vi "SMain.vi"() -> ()   [LabVIEW 2011] (continued)
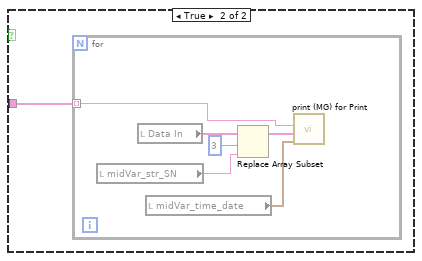
[diagram p4: hidden frame]
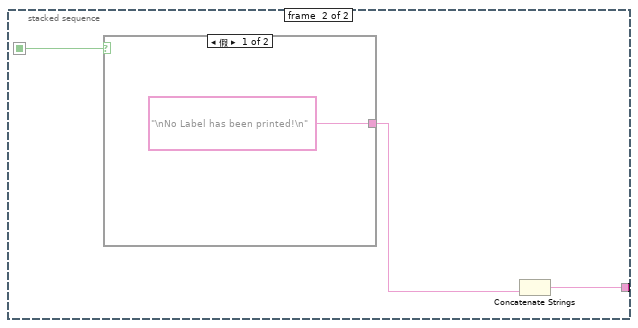
[diagram p5: hidden frame]
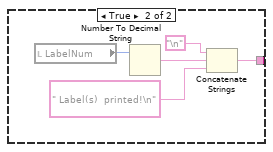
[diagram p6: hidden frame]
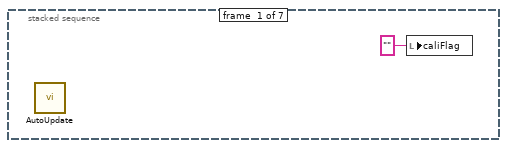
[diagram p8: hidden frame]
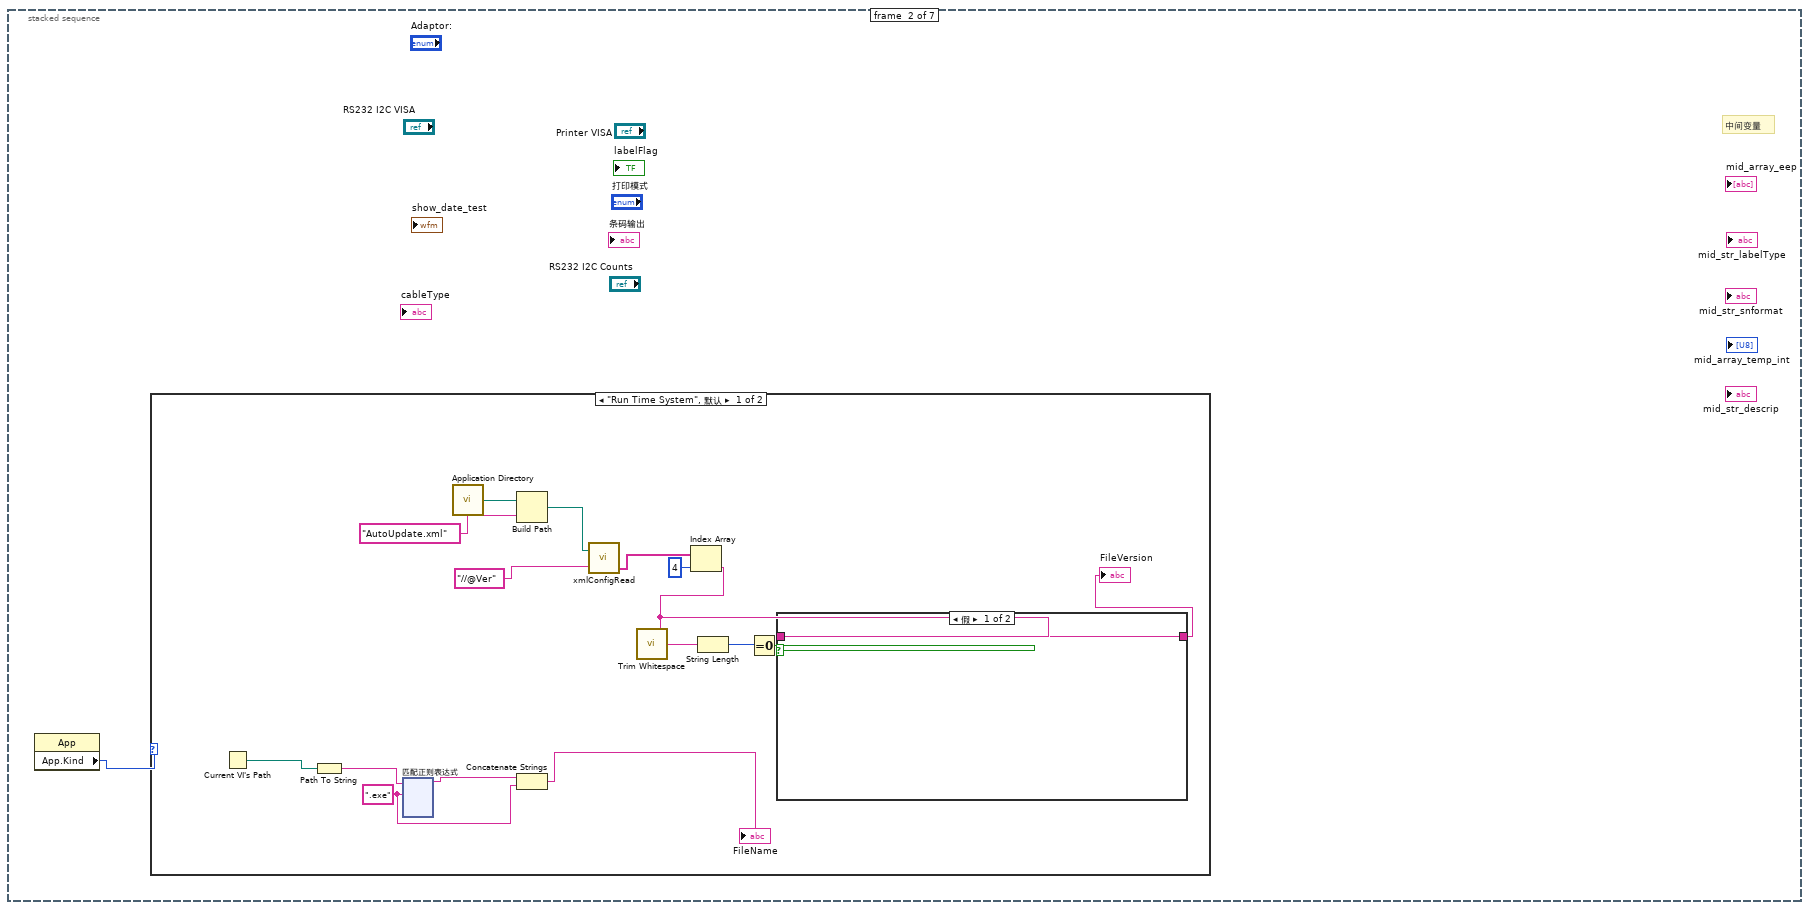
[diagram p9: hidden frame]
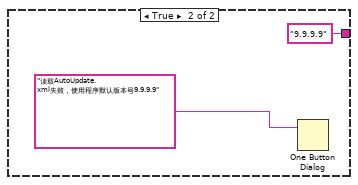
[diagram p10: hidden frame]
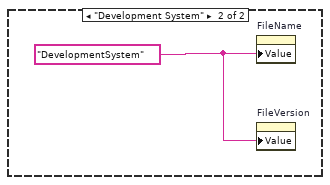
[diagram p11: hidden frame]
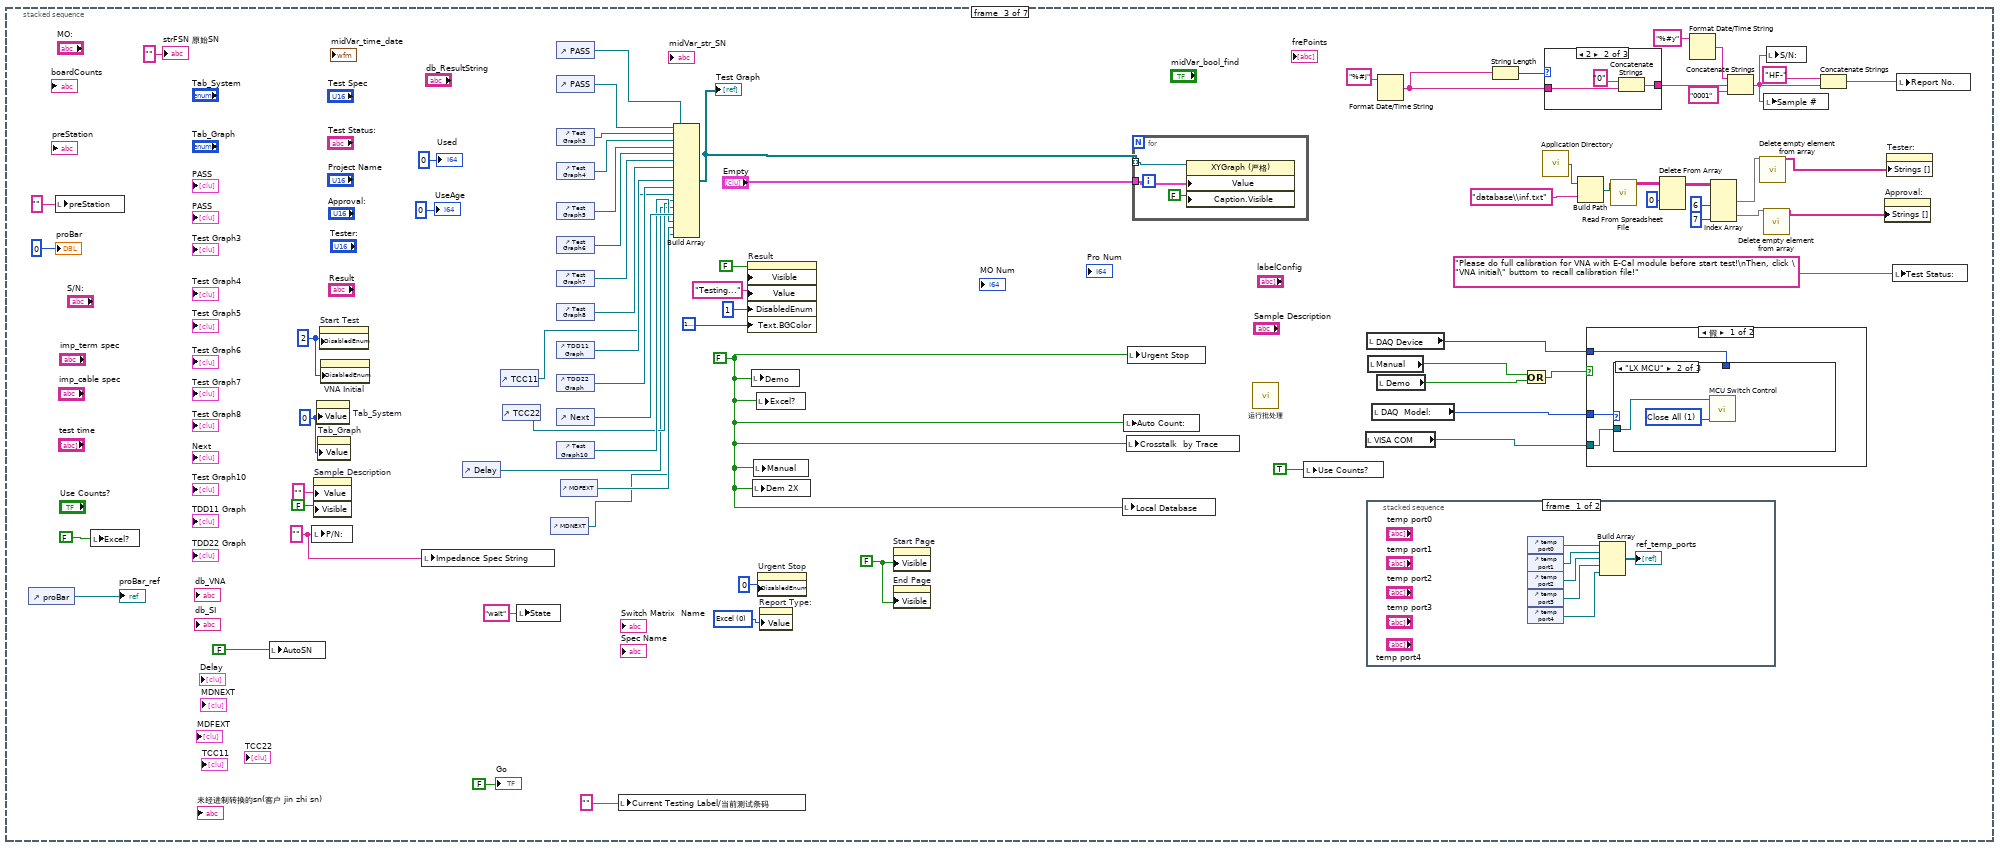
[diagram p12: hidden frame]
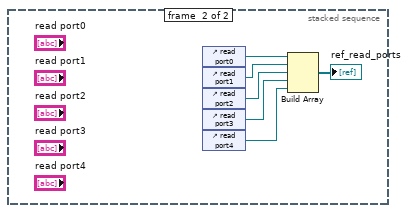
[diagram p13: hidden frame]
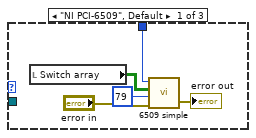
[diagram p14: hidden frame]
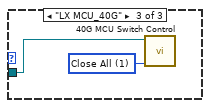
[diagram p15: hidden frame]
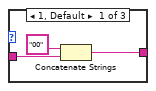
[diagram p17: hidden frame]
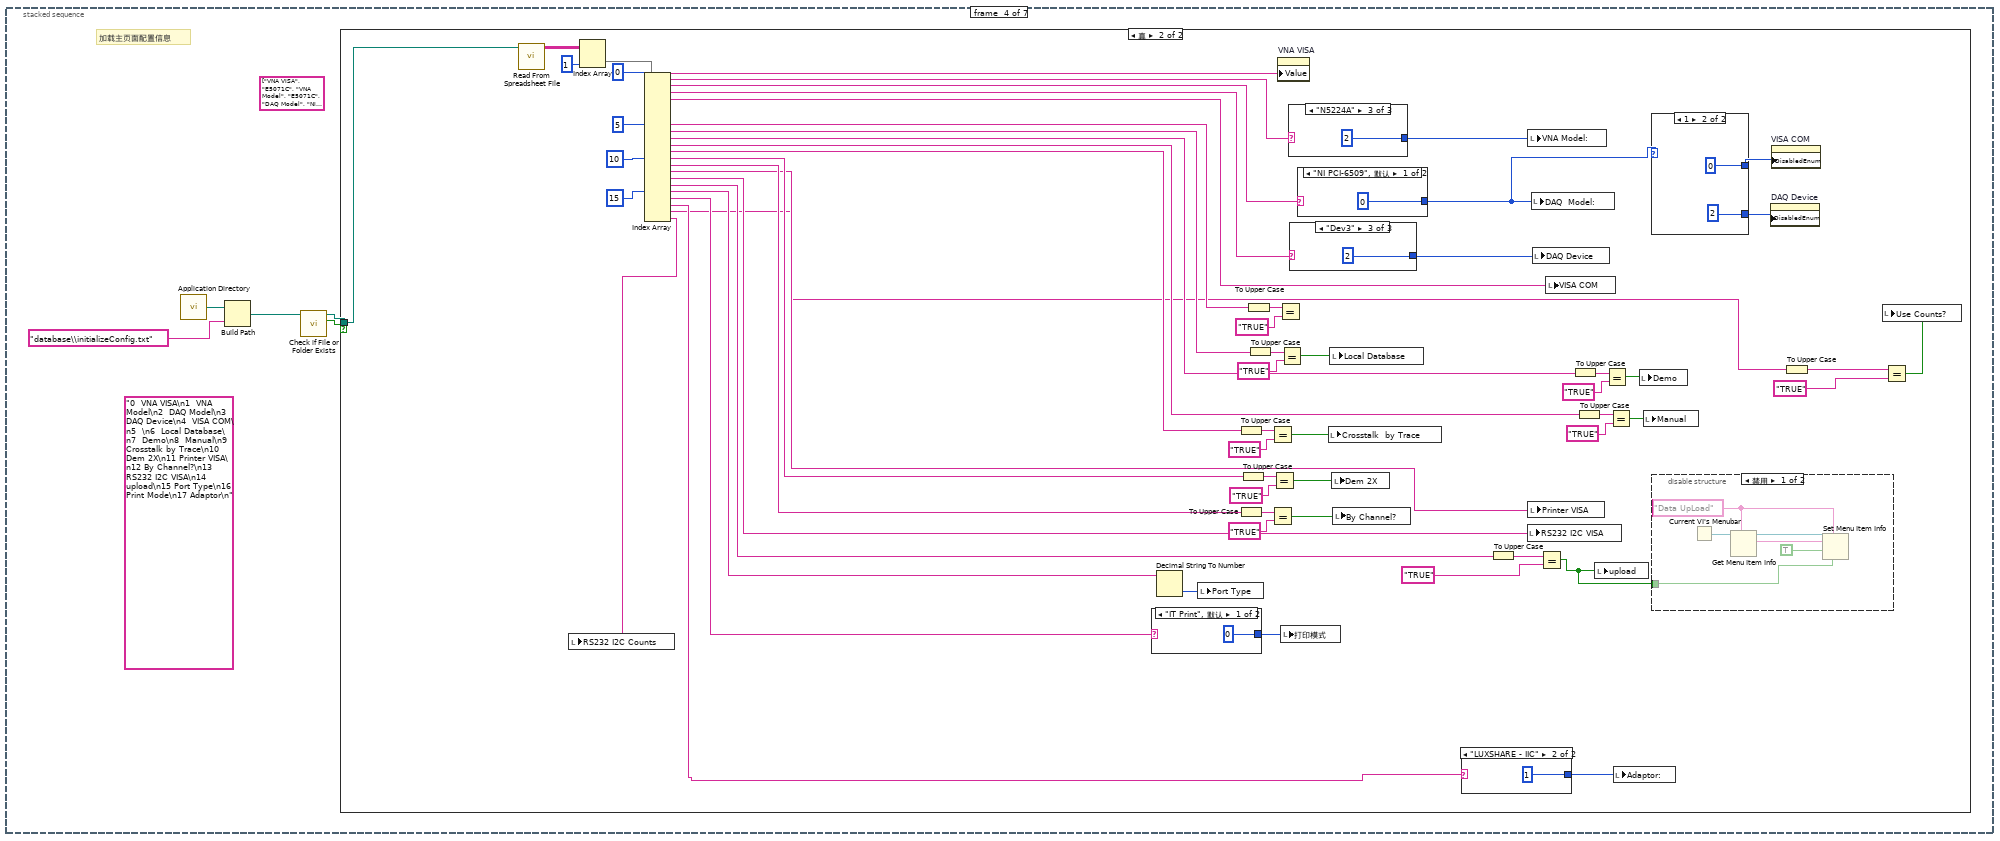
[diagram p19: hidden frame]
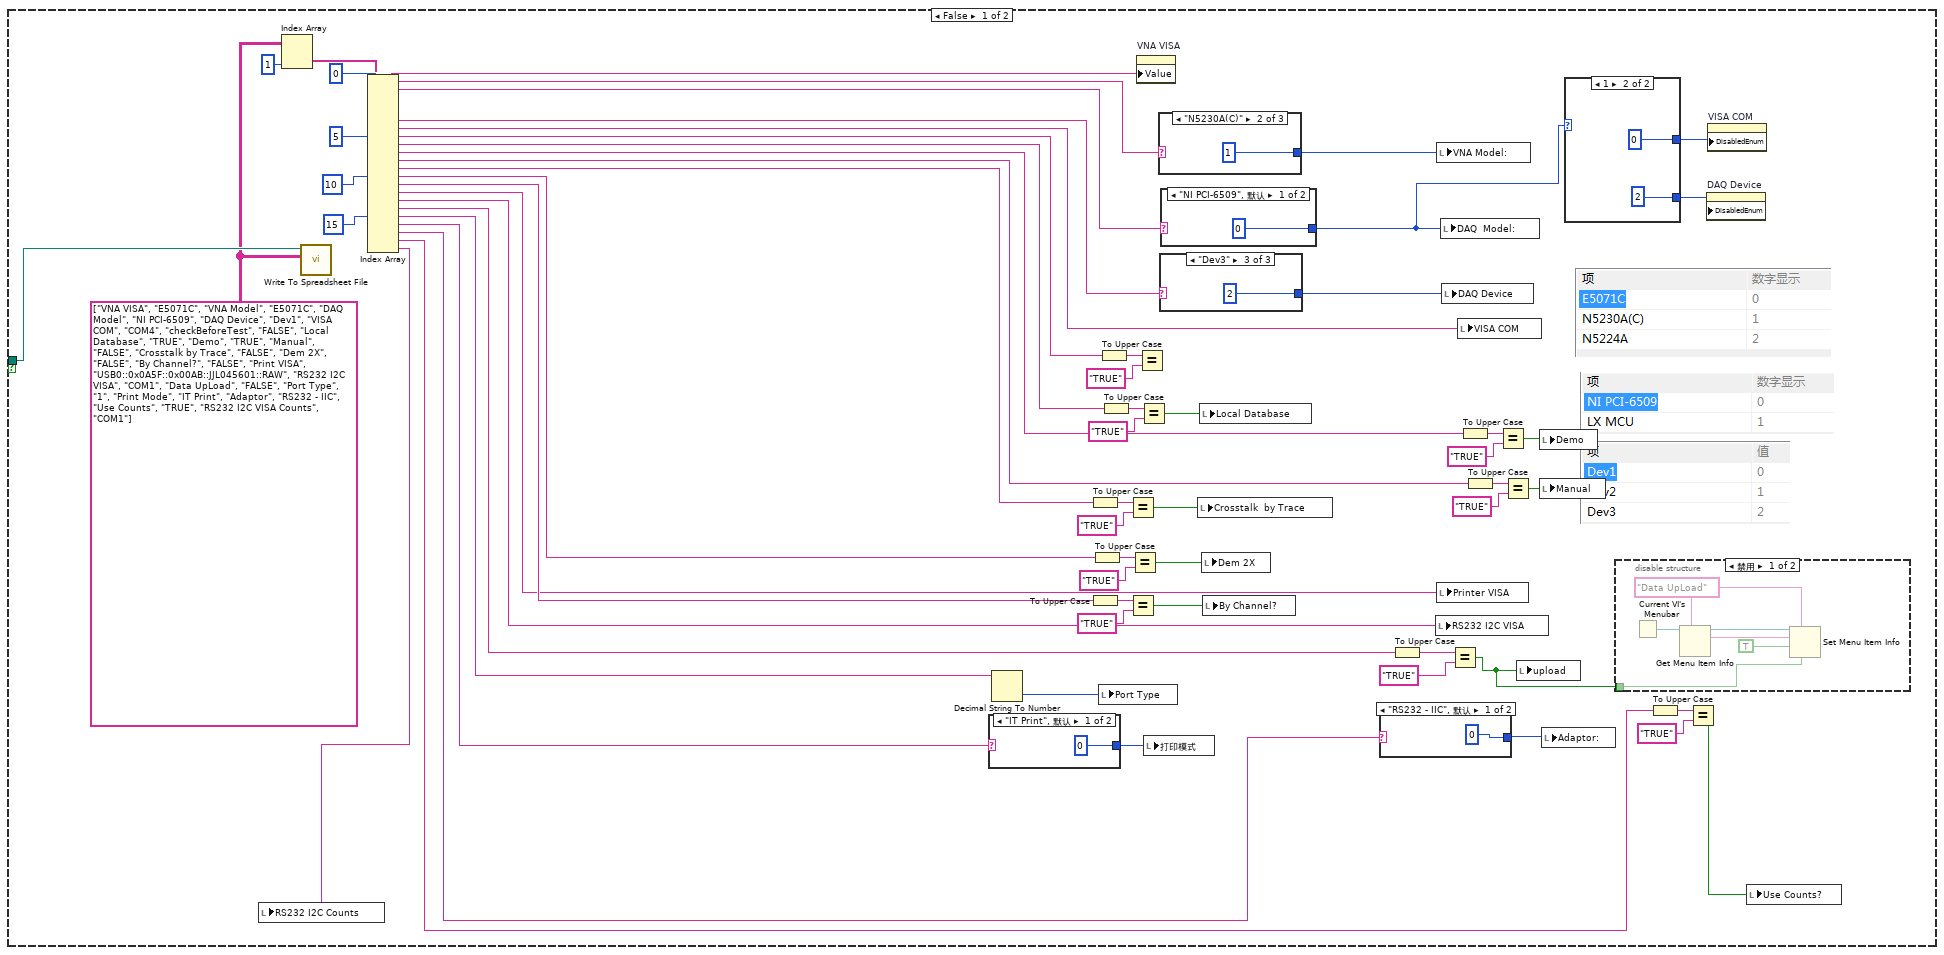
[diagram p20: hidden frame]
                        n1540 = Fract/Exp String To Number(string=w2418) -> (number=w2409:dbl)  [unwired: 3 in, 1 out]
                        n1541 = Fract/Exp String To Number(string=w2419) -> (number=w2410:dbl)  [unwired: 3 in, 1 out]
                        n1542 = Decimal String To Number(string=w2417) -> (number=w2408:i32)  [unwired: 2 in, 1 out]
                        n1543 = Spreadsheet String To Array(format string="%s" ("格式字符串"), spreadsheet string=w2404, array type (2D Dbl)=dbl[] []) -> (array=→"2X IL 2":dbl[])  [unwired: 1 in]
                        n1544 = Fract/Exp String To Number(string=w2416) -> (number=w2407:dbl)  [unwired: 3 in, 1 out]
                        n1545 = Equal?(x=w2413, y="1") -> (x = y?=w2411:bool)
                        n1546 = Fract/Exp String To Number(string=w2414) -> (number=w2406:dbl)  [unwired: 3 in, 1 out]
                        n1547 = local write "Impedance Spec String 2"(w2412) -> ()
                        n1548 = local write "Start TimeNs 2"(w2410) -> ()
                        n1549 = local write "StopTimeNs 2"(w2409) -> ()
                        n1550 = local write "Filter Risetime(ps) 2"(w2407) -> ()
                        n1551 = local write "Data Points 2"(w2408) -> ()
                        n1552 = local write "Compensation(ohm) 2"(w2406) -> ()
                        n1553 = local write "Impedance Filter 2"(w2411) -> ()
                      }
                      frame #8 {
                        n1554 = call "(0,1)to(true,false) by data.vi"("Switch data"=w2422) -> ("Switch array"=→"Switch array":bool[][])  [unwired: 2 in]
                      }
                      frame #9 {
                        w2425 = 8 ("y")
                        n1555 = disable-structure shown="禁用" {
                          frame Disabled {
                            n1556 = local read "Diff Test Item Name"() -> (w2430:string[])
                            n1557 = call "Divide Test Items.vi"("Test Item Name"=w2430) -> ()  [unwired: 9 in, 2 out]
                          }
                          frame Enabled {
                          }
                        }
                        n1558 = local read "S-Para Item List"() -> (w2423:string[])
                        n1559 = Array Size(array=w2423) -> (size(s)=w2427:i32)
                        n1560 = local read "Test Graph"() -> (w2429:refnum<vi>[])
                        n1561 = local read "Empty"() -> (w2428:cluster{"Horz Time array":dbl[], "Y":dbl[]}[])
                        n1562 = Less Or Equal?(x=w2427, y=w2425) -> (x <= y?=w2426:bool)
                        n1563 = Select(t=w2427, s=w2426, f=w2425) -> (s? t:f=w2424:i32)
                        n1564 = for {
                          tunnel: w2429 -> [w2436] mode=indexing
                          tunnel: w2428 -> [w2435]
                          tunnel: w2424 -> [w2432]
                          tunnel: w2423 -> [w2434]
                          i -> [w2431]
                          n1565 = Index Array(array=w2434, index=w2431) -> (element=w2433:string)
                          n1566 = Less?(x=w2431, y=w2432) -> (x < y?=w2437:bool)
                          n1567 = case shown="假" w2437 {
                            tunnel: w2436 -> [w2439 w2443]
                            tunnel: w2435 -> [w2438 w2442]
                            tunnel: w2433 -> [_ w2441]
                            frame False {
                              n1568 = property class="XYGraph (严格)"(reference=w2439, "Value"=w2438, "Caption.Visible"=FALSE ("标题.可见")) -> ()  [unwired: 1 in, 2 out]
                            }
                            frame True {
                              n1569 = property class="XYGraph (严格)"(reference=w2443, "Value"=w2442, "Caption.Visible"=TRUE ("标题.可见"), "Caption.Text"=w2441) -> ()  [unwired: 1 in, 2 out]
                            }
                          }
                        }
                      }
                      frame #10 {
                        n1570 = case shown="假" w2445 {
                          frame False {
                            n1571 = stacked-sequence {
                              seq-local: [_ w2447 _] -> [_ _ w2454]
                              frame #0 {
                                n1572 = local write "Test Status:"("Initializing VNA ....." ("Test Status:")) -> ()
                              }
                              frame #1 {
                                n1573 = local read "Cal File Path"() -> (w2448:string)
                                n1574 = local read "VNA Model:"() -> (w2449:enum16{"E5071C", "N5230A(C)", "N5224A"})
                                n1575 = local read "VNA VISA"() -> (w2450:refnum<visa-resource-name>)
                                n1576 = call "VNA Initial.vi"("Cal File Name Path"=w2448, "VNA Model:"=w2449, "VNA VISA"=w2450) -> ("Connect?"=w2447:bool)  [unwired: 8 in]
                              }
                              frame #2 {
                                n1577 = Select(t=0 ("索引"), s=w2454, f=2 ("索引")) -> (s? t:f=w2455:i32)
                                n1578 = property on="Start Test" class="Bool"("DisabledEnum"=w2455) -> ()  [unwired: 2 in, 2 out]
                                n1579 = property on="VNA Initial" class="Bool"("DisabledEnum"=w2455) -> ()  [unwired: 2 in, 2 out]
                                n1580 = Select(t="VNA Initialization Finished!\nPlease Slect Correct Project & Test Spec & Switch Matrix to Start Testing " ("Test Status:"), s=w2454, f="VNA Initialization Not Be Finished!\nPlease Check VNA Connection!" ("Test Status:")) -> (s? t:f=w2452:string)
                                n1581 = local write "Test Status:"(w2452) -> ()
                              }
                            }
                          }
                          frame True {
                            n1582 = property on="Start Test" class="Bool"("DisabledEnum"=0 ("索引")) -> ()  [unwired: 2 in, 2 out]
                            n1583 = local write "Test Status:"("Please do full calibration for VNA with E-Cal module before start test!\nThen, click \"VNA initial\" buttom to recall calibration file!" ("Test Status:")) -> ()
                          }
                        }
                      }
                      frame #11 {
                        (unwired) "Initializing VNA ....." ("Test Status:")
                        # "增加华为完整XML生成料号配置文件读取功能"
                        n1584 = call <vilib>:"Application Directory.vi"() -> ("Application Directory"=w2465:path)
                        n1585 = Build Path(base path=w2465, name or relative path="Database\\FigoConfig.xml") -> (appended path=w2463:path)
                        n1586 = call <vilib>:"Check if File or Folder Exists.vi"("path"=w2463) -> ("file or folder exists?"=w2462:bool, "dup path"=w2461:path)  [unwired: 8 in, 1 out]
                        n1587 = case shown="真" w2462 {
                          tunnel: w2461 -> [w2469 w2484]
                          tunnel: w2460 -> [_ w2489]
                          frame False {
                            n1588 = Path To String(path=w2469) -> (string=w2468:string)
                            n1589 = Concatenate Strings("文件" ("字符串"), w2468, "加载失败，将使用默认值" ("字符串")) -> (w2466:string)
                            n1590 = One Button Dialog(message=w2466) -> ()  [unwired: 1 in, 1 out]
                          }
                          frame True {
                            n1591 = local read "打印模式"() -> (w2487:enum16{"IT Print", "EE Print"})
                            n1592 = call "校验信息获取.vi"("料号"=w2489, "path to XML document"=w2484) -> ("校验信息"=→"校验信息":T7)  [unwired: 9 in]
                            n1593 = call "xmlConfigRead.vi"("path to XML document"=w2484, "XPath expression"="//PartNoWithFullXml/PartNo/@Name") -> ("OutParaArray"=w2488:string[])  [unwired: 2 out]
                            n1594 = local read "P/N:"() -> (w2486:string)
                            n1595 = call "xmlConfigRead.vi"("path to XML document"=w2484, "XPath expression"="//PartNoWith2X/PartNo/@Name") -> ("OutParaArray"=w2494:string[])  [unwired: 2 out]
                            n1596 = call "EEUpload.vi"("PN"=w2486, "打印模式"=w2487, "xmlConfigPath"=w2484) -> ("EEUPLOAD"=→"EEUPLOAD":bool)  [unwired: 6 in, 2 out]
                            n1597 = Search 1D Array(1D array=w2488, element=w2486) -> (index of element=w2500:i32)  [unwired: 1 in]
                            n1598 = Search 1D Array(1D array=w2494, element=w2486) -> (index of element=w2493:i32)  [unwired: 1 in]
                            n1599 = Equal?(x=w2500, y=-1) -> (x = y?=w2498:bool)
                            n1600 = Not Equal?(x=w2493, y=-1) -> (x != y?=w2491:bool)
                            "2x equalize" <- w2491
                            n1601 = case shown="假" w2491 {
                              frame False {
                                n1602 = local write "Test Status:"("ILD_15将会采用与SDD21设定方式进行计算") -> ()
                              }
                              frame True {
                                n1603 = local write "Test Status:"("ILD_15将会加上2X夹具值后进行计算") -> ()
                              }
                            }
                            n1604 = Not(x=w2498) -> (.not. x?=w2497:bool)
                            "FullXml" <- w2497
                            n1605 = case shown="真" w2497 {
                              tunnel: w2484 -> [_ w2523]
                              tunnel: w2486 -> [_ w2524]
                              frame False {
                                n1606 = local read "Test Status:"() -> (w2506:string)
                                n1607 = Concatenate Strings(w2506, "\n", "将生成精简的XML文件") -> (w2503:string)
                                n1608 = local write "Test Status:"(w2503) -> ()
                              }
                              frame True {
                                n1609 = Search and Replace String(input string="//PartNoWithFullXml/PartNo[@Name='@Name@']/@*" ("XPath expression"), search string="@Name@" ("搜索字符串"), replace string=w2524) -> (result string=w2528:string)  [unwired: 5 in, 3 out]
                                n1610 = call "xmlConfigRead.vi"("path to XML document"=w2523, "XPath expression"=w2528) -> ("OutParaArray"=w2527:string[])  [unwired: 2 out]
                                n1611 = Index Array(array=w2527, index #1=1 ("索引"), index #2=2 ("索引"), index #3=3 ("索引"), index #4=4 ("索引")) -> (element #1=w2519:string, element #2=→"PN TYpe":string, element #3=w2509:string, element #4=w2508:string)
                                n1612 = local read "Test Status:"() -> (w2514:string)
                                n1613 = To Upper Case(1:w2519) -> (0:w2520:string)
                                n1614 = Decimal String To Number(string=w2509) -> (number=→"width1":i32)  [unwired: 2 in, 1 out]
                                n1615 = Decimal String To Number(string=w2508) -> (number=→"width2":i32)  [unwired: 2 in, 1 out]
                                n1616 = Equal?(x=w2520, y="TRUE") -> (x = y?=→"auto get refer point":bool)
                                n1617 = Concatenate Strings(w2514, "\n", "将生成完整频点的XML文件的华为料号，是否生成依赖FullXML?的设定") -> (w2511:string)
                                n1618 = local write "Test Status:"(w2511) -> ()
                              }
                            }
                            n1619 = call "xmlConfigRead.vi"("path to XML document"=w2484, "XPath expression"="//UploadPara/*") -> ("OutParaArray"=w2482:string[])  [unwired: 2 out]
                            n1620 = Index Array(array=w2482) -> (element #1=w2480:string, element #2=w2479:string, element #3=w2478:string, element #4=w2477:string, element #5=w2476:string, element #6=w2475:string, element #7=w2474:string, element #8=w2472:string, element #9=w2471:string)  [unwired: 9 in]
                            n1621 = Bundle By Name(cluster=T1 {"NetCmdHW"="", "NetPathHW"="", "NetCmdCompress"="", "NetPathCompress1"="", "NetPathCompress2"="", "AlarmDisplay"="", "Synchronous"="", "NetTemppath"="", "NetLocalpath"=""} ("UploadPara"), "NetCmdHW"=w2480, "NetPathHW"=w2479, "NetCmdCompress"=w2478, "NetPathCompress1"=w2477, "NetPathCompress2"=w2476, "AlarmDisplay"=w2475, "Synchronous"=w2474, "NetTemppath"=w2472, "NetLocalpath"=w2471) -> (→"uploadPara":T1)
                            n1622 = call "createFolder.vi"("字符串"=w2472) -> ()  [unwired: 11 in]
                            n1623 = call "createFolder.vi"("字符串"=w2471) -> ()  [unwired: 11 in]
                          }
                        }
                      }
                      frame #12 {
                        n1624 = Index Array(array=w2536, index=2 ("索引")) -> (element=w2534:string)
                        n1625 = To Upper Case(1:w2534) -> (0:w2533:string)
                        n1626 = Equal?(x=w2533, y="HUAWEI") -> (x = y?=w2531:bool)
                        "PassCount?" <- w2531
                        n1627 = property on="Passed" class="DigNum (严格)"("Visible"=w2531) -> ()  [unwired: 2 in, 2 out]
                        n1628 = property on="Total" class="DigNum (严格)"("Visible"=w2531) -> ()  [unwired: 2 in, 2 out]
                        n1629 = property on="Failed" class="DigNum (严格)"("Visible"=w2531) -> ()  [unwired: 2 in, 2 out]
                        n1630 = property on="ratio" class="DigNum (严格)"("Visible"=w2531) -> ()  [unwired: 2 in, 2 out]
                        n1631 = case shown="真" w2531 {
                          tunnel: w2530 -> [_ w2548]
                          frame False {
                          }
                          frame True {
                            n1632 = Format Date/Time String(time format string (%c)="%Y%m%d" ("时间格式字符串(%c)")) -> (date/time string=w2545:string)  [unwired: 2 in]
                            n1633 = call <vilib>:"Application Directory.vi"() -> ("Application Directory"=w2551:path)
                            n1634 = Concatenate Strings("DataBase\\" ("字符串"), w2548, "\\" ("字符串"), w2545, ".xml" ("字符串")) -> (w2543:string)
                            n1635 = Build Path(base path=w2551, name or relative path=w2543) -> (appended path=w2550:path)
                            "CountXmlPath" <- w2550
                            n1636 = call <vilib>:"Check if File or Folder Exists.vi"("path"=w2550) -> ("file or folder exists?"=w2542:bool, "dup path"=w2541:path)  [unwired: 8 in, 1 out]
                            n1637 = case shown="真" w2542 {
                              tunnel: w2541 -> [w2552 w2571]
                              tunnel: [0 w2567] -> w2540
                              tunnel: [0 w2565] -> w2539
                              tunnel: [0 w2564] -> w2538
                              tunnel: [0.0 w2563] -> w2537
                              frame False {
                                n1638 = stacked-sequence {
                                tunnel: w2552 -> [w2560 w2562]
                                frame #0 {
                                n1639 = Strip Path(path=w2560) -> (stripped path=w2559:path)  [unwired: 1 out]
                                n1640 = call <vilib>:"Check if File or Folder Exists.vi"("path"=w2559) -> ("file or folder exists?"=w2558:bool, "dup path"=w2557:path)  [unwired: 8 in, 1 out]
                                n1641 = case shown="假" w2558 {
                                tunnel: w2557 -> [w2561 _]
                                frame False {
                                n1642 = Create Folder(path (use dialog)=w2561) -> ()  [unwired: 2 in, 3 out]
                                }
                                frame True {
                                }
                                }
                                }
                                frame #1 {
                                n1643 = call "xmlNodecreate.vi"("path"=w2562) -> ()  [unwired: 3 in, 1 out]
                                }
                                }
                              }
                              frame True {
                                # "增加华为完整XML生成料号配置文件读取功能"
                                n1644 = call "xmlConfigRead.vi"("path to XML document"=w2571, "XPath expression"="//FailedSN/*") -> ("OutParaArray"=w2568:string[])  [unwired: 2 out]
                                n1645 = call "xmlConfigRead.vi"("path to XML document"=w2571, "XPath expression"="//PassedSN/*") -> ("OutParaArray"=w2569:string[])  [unwired: 2 out]
                                n1646 = Array Size(array=w2569) -> (size(s)=w2567:i32)
                                n1647 = Array Size(array=w2568) -> (size(s)=w2565:i32)
                                n1648 = Add(x=w2565, y=w2567) -> (x+y=w2564:i32)
                                n1649 = Equal To 0?(x=w2564) -> (x = 0?=w2566:bool)
                                n1650 = case shown="假" w2566 {
                                tunnel: w2565 -> [w2577 _]
                                tunnel: w2564 -> [w2576 _]
                                tunnel: [w2573 0.0] -> w2563
                                frame False {
                                n1651 = Divide(x=w2577, y=w2576) -> (x/y=w2575:dbl)
                                n1652 = Multiply(x=w2575, y=100.0) -> (x*y=w2573:dbl)
                                }
                                frame True {
                                }
                                }
                              }
                            }
                            "Total" <- w2538
                            "Passed" <- w2540
                            "Failed" <- w2539
                            "ratio" <- w2537
                          }
                        }
                      }
                      frame #13 {
                        n1653 = call "getDebugMode.vi"() -> ("debugMode"=w2579:bool)  [unwired: 11 in]
                        n1654 = case shown="真" w2579 {
                          frame False {
                          }
                          frame True {
                            n1655 = One Button Dialog(message="当前模式为debug模式，仅可用于调试用\n请注意" ("消息")) -> ()  [unwired: 1 in, 1 out]
                          }
                        }
                        n1656 = local read "SystemMode"() -> (w2583:string)
                        n1657 = local read "DB1"() -> (w2582:T8)
                        n1658 = call "checkCalistatus.vi"("DBSet"=w2582, "SystemMode"=w2583) -> ("calibrated?"=w2581:bool)  [unwired: 9 in]
                        n1659 = Or(x=w2581, y=w2579) -> (x .or. y?=w2580:bool)
                        n1660 = case shown="真" w2580 {
                          frame False {
                            n1661 = local read "caliDataSelect"() -> (w2585:bool)
                            n1662 = case shown="真" w2585 {
                              frame False {
                                n1663 = One Button Dialog(message="请先选择sampleNo" ("消息")) -> ()  [unwired: 1 in, 1 out]
                                n1664 = property on="Start Test" class="Bool"("DisabledEnum"=T17."Disabled and Grayed Out" ("禁用")) -> ()  [unwired: 2 in, 2 out]
                              }
                              frame True {
                                n1665 = property on="Start Test" class="Bool"("BoolText.Text"="Calibrate" ("布尔文本.文本")) -> ()  [unwired: 2 in, 2 out]
                                n1666 = property on="Start Test" class="Bool"("DisabledEnum"=T17."Enabled" ("禁用")) -> ()  [unwired: 2 in, 2 out]
                                n1667 = One Button Dialog(message="该测试机台当日未校验，测试前需要校验" ("消息")) -> ()  [unwired: 1 in, 1 out]
                                "caliFlag" <- "cali"
                              }
                            }
                          }
                          frame True {
                            n1668 = property on="Start Test" class="Bool"("BoolText.Text"="START TEST" ("布尔文本.文本")) -> ()  [unwired: 2 in, 2 out]
                            n1669 = One Button Dialog(message="该机台已经通过校验，可以开始测试") -> ()  [unwired: 1 in, 1 out]
                            n1670 = local write "caliFlag"("" ("caliFlag")) -> ()
                          }
                        }
                      }
                      frame #14 {
                      }
                    }
                  }
                }
              }
              event "P/N:": Key Down? {
                n1671 = event-data() -> ("Char"=w2596:i16)  [unwired: 1 in, 8 out]
                n1672 = call "aToAchar.vi"("old char"=w2596) -> ("new char"=w2595:dbl)
                n1673 = event-data("Char"=w2595) -> ()  [unwired: 6 in, 1 out]
              }
              event "MO:": Key Down? {
                n1674 = event-data() -> ("Char"=w2597:i16)  [unwired: 1 in, 8 out]
                n1675 = call "aToAchar.vi"("old char"=w2597) -> ("new char"=w2598:dbl)
                n1676 = event-data("Char"=w2598) -> ()  [unwired: 6 in, 1 out]
              }
              event "VNA Initial": Value Change {
                n1677 = event-data() -> ()  [unwired: 1 in, 5 out]
              }
              event Panel Close? {
                n1678 = event-data() -> ()  [unwired: 1 in, 3 out]
                n1679 = call <vilib>:"Application Directory.vi"() -> ("Application Directory"=w2602:path)
                n1680 = Build Path(base path=w2602, name or relative path="Database" ("名称或相对路径")) -> (appended path=w2605:path)
                n1681 = Build Path(base path=w2605, name or relative path="FigoConfig.xml" ("名称或相对路径")) -> (appended path=w2601:path)
                n1682 = call <vilib>:"Check if File or Folder Exists.vi"("path"=w2601) -> ("file or folder exists?"=w2599:bool, "dup path"=w2600:path)  [unwired: 8 in, 1 out]
                n1683 = case shown="真" w2599 {
                  tunnel: w2600 -> [_ w2611]
                  frame False {
                  }
                  frame True {
                    n1684 = local read "P/N:"() -> (w2627:string)
                    n1685 = local read "MO:"() -> (w2628:string)
                    n1686 = Path To String(path=w2611) -> (string=w2614:string)
                    n1687 = call-poly <vilib>:"Load.vi"("path to XML document"=w2611) -> ("DOM document out"=w2623:refnum<k20>, "error out"=w2621:errorcluster)  [unwired: 12 in, 1 out]
                    n1688 = Build Array(w2627, w2628) -> (w2626:string[])
                    n1689 = call <vilib>:"Get All Matched Nodes.vi"("error in (no error)"=w2621, "XPath expression"="//LastPartNo/*", "node in"=w2623) -> ("error out"=w2620:errorcluster, "node result array"=w2625:refnum<k20>[], "node out"=w2622:refnum<k20>)  [unwired: 6 in]
                    n1690 = for {
                      tunnel: w2625 -> [w2633] mode=indexing
                      tunnel: w2626 -> [w2630] mode=indexing
                      shift-right: [w2631] -> w2619
                      shift-left: w2620 -> [w2632]
                      n1691 = call <vilib>:"Set Node Text Content.vi"("error in (no error)"=w2632, "newValue"=w2630, "node in"=w2633) -> ("error out"=w2631:errorcluster)  [unwired: 6 in, 2 out]
                    }
                    n1692 = call <vilib>:"Save.vi"("error in (no error)"=w2619, "XML file path"=w2611, "DOM document in"=w2622) -> ("error out"=w2608:errorcluster)  [unwired: 6 in, 2 out]
                    n1693 = Search and Replace String(replace all?=TRUE ("替换全部？(F)"), input string=w2614, search string="\\" ("搜索字符串"), replace string="\\\\" ("替换字符串(\"\")"), error in=w2608) -> (result string=w2609:string, error out=w2607:errorcluster)  [unwired: 3 in, 2 out]
                    n1694 = constructor class="Operate"(error in=w2607) -> (reference out=w2616:refnum<k24>, error out=w2615:errorcluster)  [unwired: 2 in, 1 out]
                    n1695 = invoke class="Operate" method="xmlFormat"(reference=w2616, error in=w2615, "strFilePath"=w2609) -> (error out=w2606:errorcluster)  [unwired: 1 in, 3 out]
                    n1696 = Unbundle By Name(w2606) -> ("status"=w2618:bool, "source"=w2617:string)  [unwired: 1 out]
                    n1697 = case shown="真" w2618 {
                      tunnel: w2617 -> [_ w2629]
                      frame False {
                      }
                      frame True {
                        n1698 = One Button Dialog(message=w2629) -> ()  [unwired: 1 in, 1 out]
                      }
                    }
                  }
                }
                n1699 = event-data() -> ()  [unwired: 2 in, 1 out]
              }
            }
          }
        }
      }
      n1700 = while {
        stop <- w589 stop-if-true
        n1701 = local read "Urgent Stop"() -> (w589:bool)
        n1702 = Wait (ms)(milliseconds to wait=u32 50 ("等待时间（毫秒）")) -> ()  [unwired: 1 out]
        n1703 = global write "全局.vi" "manual stop"(w589) -> ()
      }
    }
  }
  n1704 = disable-structure shown="禁用" {
    frame Disabled {
      n1705 = local read "midVar_time_date"() -> (w2637:timestamp)
      n1706 = local read "midVar_str_SN"() -> (w2638:string)
      n1707 = local read "Printer VISA"() -> (w2642:refnum<visa-resource-name>)
      n1708 = local read "Label Type"() -> (w2636:string[])
      n1709 = local read "LabelNum"() -> (w2634:i32)
      n1710 = local read "Data In"() -> (w2635:string[])
      n1711 = local read "PRINT"() -> (w2644:refnum<k24>)
      n1712 = local read "打印模式"() -> (w2639:enum16{"IT Print", "EE Print"})
      n1713 = local read "SN"() -> (w2643:refnum<k24>)
      n1714 = call "打标签模式选择.vi"("LabelNum"=w2634, "Printer VISA"=w2642, "Data In"=w2635, "Label Type"=w2636, "midVar_time_date"=w2637, "打印模式"=w2639, "midVar_str_SN"=w2638, "引用"=w2643, "PRINT"=w2644) -> ("labelFlag"=w2640:bool, "条码输出"=w2641:string)  [unwired: 7 in, 2 out]
      n1715 = local write "labelFlag"(w2640) -> ()
      n1716 = local write "条码输出"(w2641) -> ()
    }
    frame Enabled {
    }
  }
  n1717 = disable-structure shown="禁用" {
    frame Disabled {
      n1718 = stacked-sequence {
        seq-local: [w2645 _] -> [_ w2658]
        tunnel: [_ w2659] -> _
        frame #0 {
          n1719 = local read "Label Type"() -> (w2648:string[])
          n1720 = local read "LabelNum"() -> (w2647:i32)
          n1721 = Array Size(array=w2648) -> (size(s)=w2646:i32)
          n1722 = Equal?(x=w2647, y=w2646) -> (x = y?=w2645:bool)
          n1723 = case shown="假" w2645 {
            tunnel: w2648 -> [_ w2650]
            frame False {
              n1724 = One Button Dialog(message="Label数目的输入和\nLabel的类型数量不匹配！\n拒绝打印！\n需要修改Project信息" ("消息")) -> ()  [unwired: 1 in, 1 out]
            }
            frame True {
              n1725 = for {
                tunnel: w2650 -> [w2654] mode=indexing
                n1726 = local read "midVar_str_SN"() -> (w2651:string)
                n1727 = local read "Data In"() -> (w2657:string[])
                n1728 = local read "midVar_time_date"() -> (w2653:timestamp)
                n1729 = Replace Array Subset(array=w2657, new element=w2651, index=3 ("索引")) -> (w2655:string[])
                n1730 = call "print (MG) for Print.vi"("input_time_date"=w2653, "Data in"=w2655, "Label Type"=w2654) -> ("条码输出 2"=w2652:string)  [unwired: 7 in, 1 out]
              }
            }
          }
        }
        frame #1 {
          n1731 = case shown="假" w2658 {
            tunnel: ["\nNo Label has been printed!\n" w2662] -> w2660
            frame False {
            }
            frame True {
              n1732 = local read "LabelNum"() -> (w2666:i32)
              n1733 = Number To Decimal String(number=w2666) -> (decimal integer string=w2665:string)  [unwired: 1 in]
              n1734 = Concatenate Strings("\n", w2665, " Label(s)  printed!\n") -> (w2662:string)
            }
          }
          n1735 = Concatenate Strings(w2660) -> (w2659:string)  [unwired: 1 in]
        }
      }
    }
    frame Enabled {
    }
  }
  n1736 = disable-structure shown="禁用" {
    frame Disabled {
    }
    frame Enabled {
    }
  }
